vi "IR Opo Main.vi"() -> ()   [LabVIEW 2016] (continued)
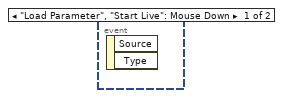
[diagram p2: hidden frame]
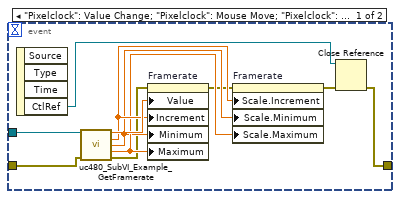
[diagram p3: hidden frame]
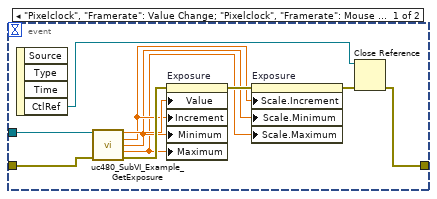
[diagram p4: hidden frame]
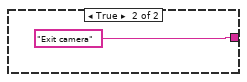
[diagram p5: hidden frame]
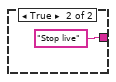
[diagram p6: hidden frame]
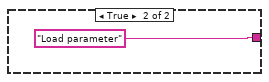
[diagram p7: hidden frame]
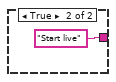
[diagram p8: hidden frame]
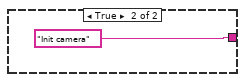
[diagram p9: hidden frame]
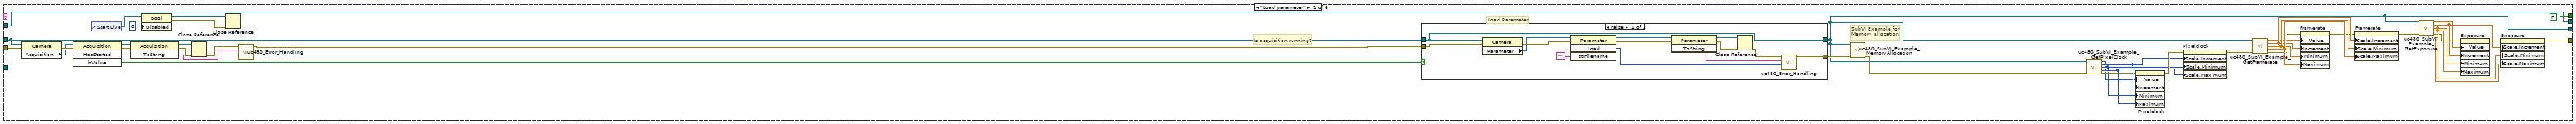
[diagram p10: hidden frame]
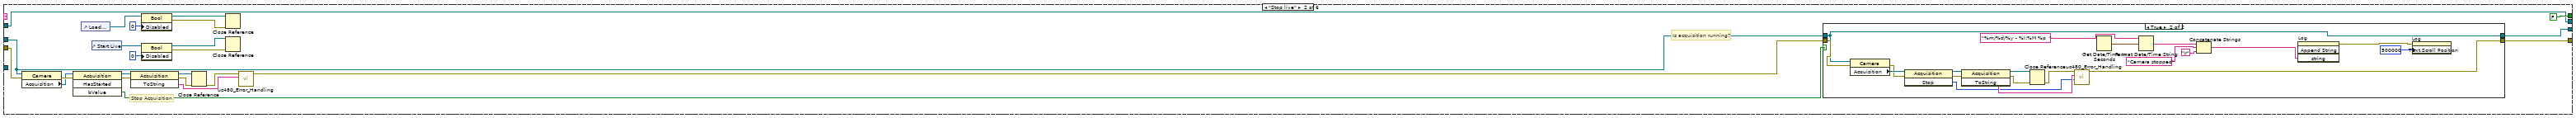
[diagram p12: hidden frame]
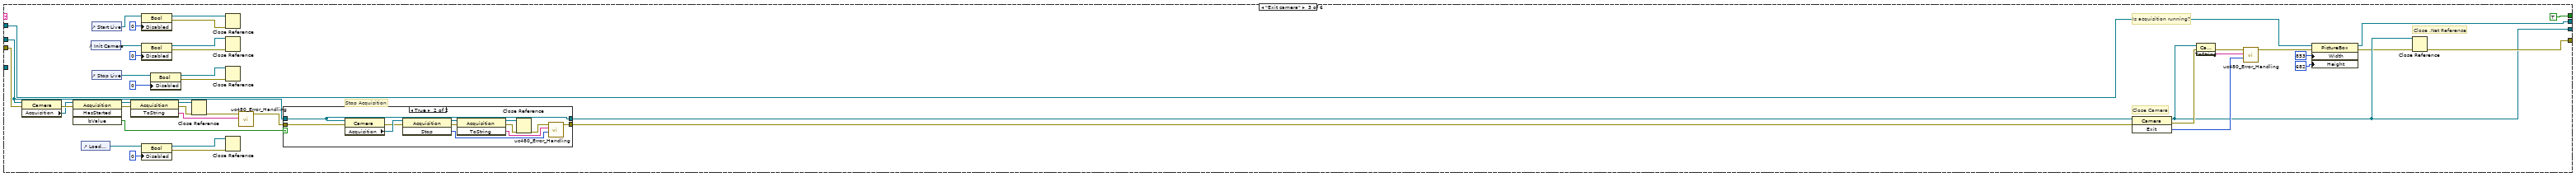
[diagram p14: hidden frame]
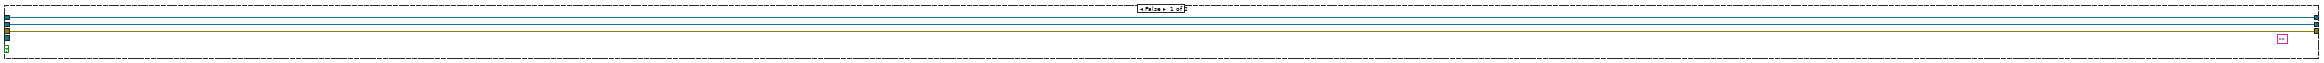
[diagram p16: hidden frame]
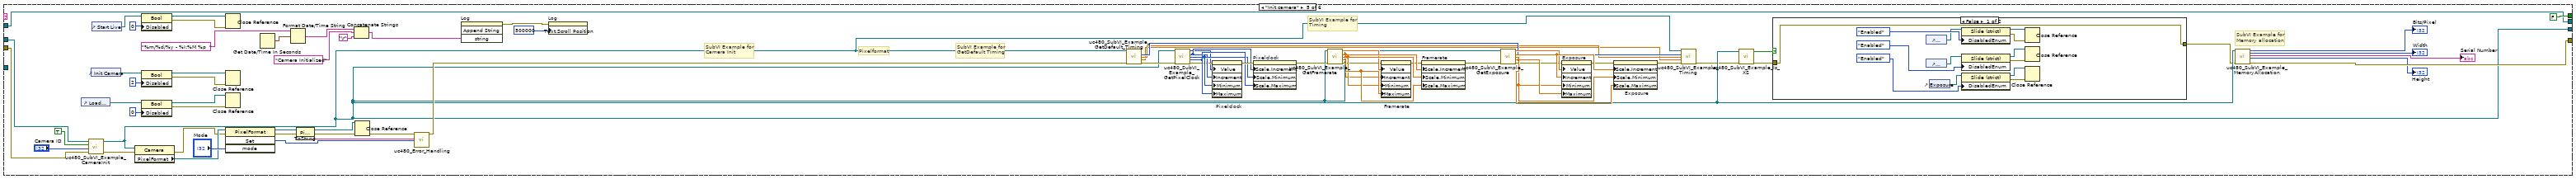
[diagram p18: hidden frame]
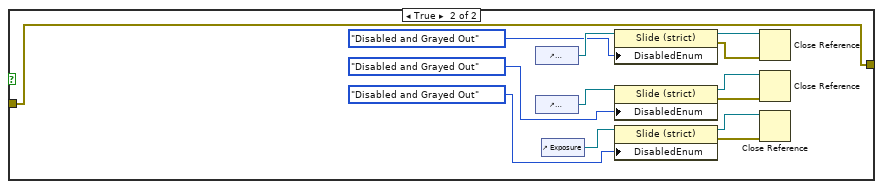
[diagram p19: hidden frame]
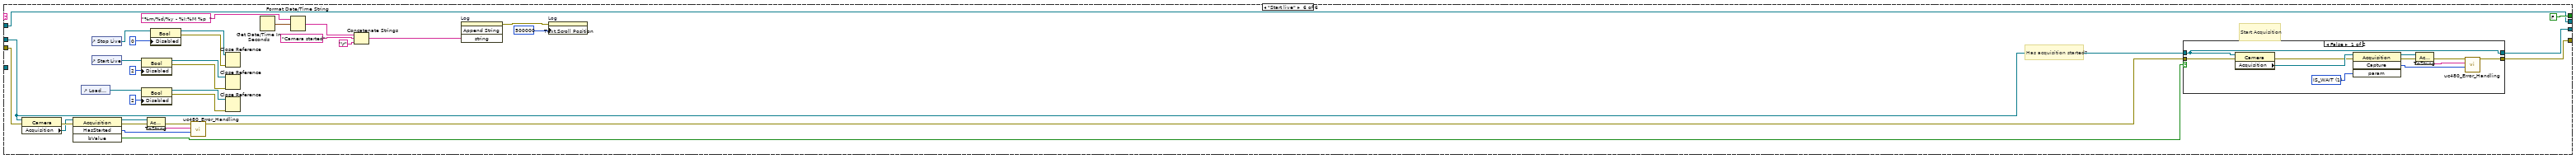
[diagram p20: hidden frame]
            n585 = call <vilib>:"Check if File or Folder Exists.vi"("path"=w1404) -> ("file or folder exists?"=w1403:bool, "dup path"=w1402:path)  [unwired: 8 in, 1 out]
            n586 = case shown="True" w1403 {
              tunnel: w1402 -> [w1414 w1415]
              tunnel: [w1413 w1415] -> w1401
              frame False {
                n587 = Create Folder(path (use dialog)=w1414) -> (created path=w1413:path)  [unwired: 2 in, 2 out]
              }
              frame True {
              }
            }
            n588 = Get Date/Time In Seconds() -> (seconds since 1Jan1904=w1398:timestamp)
            n589 = Format Date/Time String(time format string (%c)="%d%m%y %I-%M %p ", seconds (now)=w1398) -> (date/time string=w1397:string)  [unwired: 1 in]
            n590 = Concatenate Strings(w1397, " - saved ROI.tiff" ("string")) -> (w1395:string)
            n591 = Build Path(base path=w1401, name or relative path=w1395) -> (appended path=w1400:path)
            n592 = call-poly "IMAQ Write File 2"("File Path"=w1400, "Image"=w1408) -> ()  [unwired: 8 in, 2 out]
          }
        }
      }
      event "Load ROI": Value Change {
        n593 = event-data() -> ()  [unwired: 1 in, 6 out]
        n594 = case shown="True" "Load ROI" {
          frame False {
          }
          frame True {
            n595 = call "File Dialog"("prompt"="Select an ROI file..." ("pattern label"), "pattern (all files)"="*.jpg;*.bmp;*.jpeg;*.tif;*.tiff;*.png", "pattern label"="ROI files") -> ("selected path"=w1417:path, "cancelled"=w1418:bool)  [unwired: 9 in, 2 out]
            n596 = case shown="False" w1418 {
              tunnel: w1417 -> [w1429 _]
              frame False {
                n597 = call "IMAQ Create"("Image Name"="untitled") -> ("New Image"=w1431:T2)  [unwired: 4 in, 1 out]
                n598 = call "IMAQ ReadFile"("File Path"=w1429, "Image"=w1431) -> ("Image Out"=w1430:T2)  [unwired: 5 in, 4 out]
                n599 = call "IMAQ MaskToROI"("Image"=w1430) -> ("ROI Descriptor"=w1422:T13)  [unwired: 6 in, 2 out]
                n600 = Unbundle By Name(w1422) -> ("Contours"=w1427:T14)  [unwired: 1 out]
                n601 = Index Array(array=w1427) -> (element=w1428:T15)  [unwired: 1 in]
                n602 = Bundle By Name(cluster=w1428, "Type"=u32 6) -> (w1426:T15)
                n603 = Replace Array Subset(array=w1427, new element=w1426) -> (w1425:T14)  [unwired: 1 in]
                n604 = Bundle By Name(cluster=w1422, "Contours"=w1425) -> (w1423:T13)
                n605 = property on="Source" class="ImageControl"("ROI"=w1423) -> ()  [unwired: 2 in, 2 out]
              }
              frame True {
              }
            }
          }
        }
      }
      event "Axes Manual Control": Value Change {
        n606 = event-data() -> ()  [unwired: 1 in, 6 out]
        n607 = case shown="True" "Axes Manual Control" {
          tunnel: w1435 -> [_ w1447]
          tunnel: w1434 -> [_ w1446]
          tunnel: w1433 -> [_ w1445]
          frame False {
          }
          frame True {
            n608 = flat-sequence {
              tunnel: w1447 -> [w1457]
              tunnel: w1446 -> [w1456]
              tunnel: w1445 -> [w1455]
              tunnel: [w1457] -> w1444
              tunnel: [w1456] -> w1443
              tunnel: [w1455] -> w1442
              tunnel: [w1454] -> w1441
              tunnel: [w1453] -> w1440
              tunnel: [w1452] -> w1439
              tunnel: [w1451] -> w1438
              tunnel: w1444 -> [w1500]
              tunnel: w1443 -> [w1499]
              tunnel: w1442 -> [w1498]
              tunnel: w1441 -> [w1493]
              tunnel: w1440 -> [w1492]
              tunnel: w1439 -> [w1483]
              tunnel: w1438 -> [w1482]
              frame #0 {
                n609 = call <userlib>:"Open TCP-IP.vi"("IP address"=w1457) -> ("error out"=w1449:errorcluster, "Connection ID"=w1458:T9)  [unwired: 8 in, 1 out]
                n610 = call <vilib>:"Simple Error Handler.vi"("error in (no error)"=w1449) -> ("error?"=w1448:bool, "error out"=w1450:errorcluster)  [unwired: 4 in, 3 out]
                n611 = case shown="True" w1448 {
                  tunnel: w1458 -> [w1473 _]
                  tunnel: w1450 -> [w1472 _]
                  tunnel: w1456 -> [w1469 _]
                  tunnel: w1455 -> [w1468 _]
                  tunnel: [w1467 w1477] -> w1454
                  tunnel: [w1466 w1477] -> w1453
                  tunnel: [w1462 w1476] -> w1452
                  tunnel: [w1461 w1476] -> w1451
                  frame False {
                    n612 = call "Get Stages Status.vi"("error in (no error)"=w1472, "Group Name (250 c max)"=w1469, "connection ID in"=w1473) -> ("error out"=w1471:errorcluster, "XPS error out"=w1470:errorcluster, "Group Status String"=w1466:string, "connection ID out"=w1465:T9, "Status"=w1461:i32)  [unwired: 4 in]
                    n613 = call "Get Stages Status.vi"("error in (no error)"=w1471, "XPS error in (no error)"=w1470, "Group Name (250 c max)"=w1468, "connection ID in"=w1465) -> ("error out"=w1475:errorcluster, "XPS error out"=w1464:errorcluster, "Group Status String"=w1467:string, "connection ID out"=w1474:T9, "Status"=w1462:i32)  [unwired: 3 in]
                    n614 = call <vilib>:"Simple Error Handler.vi"("error source (\" \")"="Axis manual control check" ("error source (\" \")"), "error in (no error)"=w1464) -> ()  [unwired: 3 in, 5 out]
                    n615 = call <userlib>:"Close TCP-IP.vi"("error in (no error)"=w1475, "connection ID in"=w1474) -> ("Error out"=w1463:errorcluster)  [unwired: 9 in]
                    n616 = call <vilib>:"Simple Error Handler.vi"("error source (\" \")"="TCP close Axis manual control check" ("error source (\" \")"), "error in (no error)"=w1463) -> ()  [unwired: 3 in, 5 out]
                  }
                  frame True {
                    w1476 = 0
                    w1477 = ""
                  }
                }
              }
              frame #1 {
                w1486 = 47 ("y")
                w1487 = "Ready"
                n617 = String Subset(string=w1492, offset (0)=0, length (rest)=5 ("length (rest)")) -> (substring=w1489:string)
                n618 = String Subset(string=w1493, offset (0)=0, length (rest)=5 ("length (rest)")) -> (substring=w1488:string)
                n619 = Equal?(x=w1489, y=w1487) -> (x = y?=w1490:bool)
                n620 = Equal?(x=w1487, y=w1488) -> (x = y?=w1491:bool)
                n621 = Equal?(x=w1486, y=w1482) -> (x = y?=w1484:bool)
                n622 = Equal?(x=w1483, y=w1486) -> (x = y?=w1485:bool)
                n623 = And(x=w1485, y=w1484) -> (x .and. y?=w1479:bool)
                n624 = And(x=w1490, y=w1491) -> (x .and. y?=w1480:bool)
                n625 = Not(x=w1479) -> (.not. x?=w1478:bool)
                n626 = And(x=w1480, y=w1478) -> (x .and. y?=w1481:bool)
                n627 = case shown="True" w1481 {
                  tunnel: w1500 -> [_ w1506]
                  tunnel: w1499 -> [_ w1505]
                  tunnel: w1498 -> [_ w1504]
                  tunnel: w1478 -> [w1501 _]
                  frame False {
                    n628 = case shown="False" w1501 {
                      frame False {
                        n629 = One Button Dialog(message="One or more axis already in jogging position") -> ()  [unwired: 1 in, 1 out]
                      }
                      frame True {
                        n630 = One Button Dialog(message="Axes are not ready") -> ()  [unwired: 1 in, 1 out]
                      }
                    }
                  }
                  frame True {
                    n631 = call "XPS_LTA_HS_Jogger.vi"("Axis 2"=w1504, "Axis 1"=w1505, "Controller Address"=w1506) -> ()  [unwired: 8 in]
                  }
                }
              }
            }
          }
        }
      }
      event "Home Axes": Value Change {
        n632 = event-data() -> ()  [unwired: 1 in, 6 out]
        n633 = flat-sequence {
          tunnel: w1513 -> [w1519]
          tunnel: w1514 -> [w1520]
          tunnel: w1515 -> [w1521]
          tunnel: "Home Axes" -> [w1522]
          tunnel: [w1522] -> w1511
          tunnel: [w1521] -> w1510
          tunnel: [w1520] -> w1509
          tunnel: [w1519] -> w1508
          tunnel: [w1518] -> w1507
          tunnel: [w1526] -> w1512
          tunnel: w1511 -> [w1524]
          tunnel: w1510 -> [w1529]
          tunnel: w1509 -> [w1527]
          tunnel: w1508 -> [w1528]
          tunnel: w1507 -> [w1525]
          tunnel: [w1608] -> w1516
          tunnel: w1512 -> [w1607]
          frame #0 {
            n634 = call "Display Message to User"() -> ("OK"=w1518:bool)  [unwired: 10 in, 1 out]
          }
          frame #1 {
            n635 = And(x=w1524, y=w1525) -> (x .and. y?=w1523:bool)
            n636 = case shown="True" w1523 {
              tunnel: w1529 -> [_ w1545]
              tunnel: w1527 -> [_ w1546]
              tunnel: w1528 -> [_ w1543]
              tunnel: w1527 -> [_ w1544]
              tunnel: [FALSE w1536] -> w1526
              frame False {
              }
              frame True {
                w1542 = 47 ("y")
                w1558 = "Ready"
                n637 = call <userlib>:"Open TCP-IP.vi"("IP address"=w1545) -> ("error out"=w1531:errorcluster, "Connection ID"=w1549:T9)  [unwired: 8 in, 1 out]
                n638 = call <vilib>:"Simple Error Handler.vi"("error in (no error)"=w1531) -> ("error?"=w1533:bool, "error out"=w1532:errorcluster)  [unwired: 4 in, 3 out]
                n639 = case shown="False" w1533 {
                  tunnel: w1532 -> [w1572 _]
                  tunnel: w1549 -> [w1571 _]
                  tunnel: [w1568 w1577] -> w1548
                  tunnel: [w1567 w1577] -> w1547
                  tunnel: w1546 -> [w1566 _]
                  tunnel: w1543 -> [w1565 _]
                  tunnel: [w1562 w1576] -> w1541
                  tunnel: [w1561 w1576] -> w1540
                  frame False {
                    n640 = call "Get Stages Status.vi"("error in (no error)"=w1572, "Group Name (250 c max)"=w1566, "connection ID in"=w1571) -> ("error out"=w1573:errorcluster, "XPS error out"=w1574:errorcluster, "Group Status String"=w1568:string, "connection ID out"=w1575:T9, "Status"=w1561:i32)  [unwired: 4 in]
                    n641 = call "Get Stages Status.vi"("error in (no error)"=w1573, "XPS error in (no error)"=w1574, "Group Name (250 c max)"=w1565, "connection ID in"=w1575) -> ("error out"=w1569:errorcluster, "XPS error out"=w1564:errorcluster, "Group Status String"=w1567:string, "connection ID out"=w1570:T9, "Status"=w1562:i32)  [unwired: 3 in]
                    n642 = call <vilib>:"Simple Error Handler.vi"("error source (\" \")"="home axis check" ("error source (\" \")"), "error in (no error)"=w1564) -> ()  [unwired: 3 in, 5 out]
                    n643 = call <userlib>:"Close TCP-IP.vi"("error in (no error)"=w1569, "connection ID in"=w1570) -> ("Error out"=w1563:errorcluster)  [unwired: 9 in]
                    n644 = call <vilib>:"Simple Error Handler.vi"("error source (\" \")"="TCP close home axis check" ("error source (\" \")"), "error in (no error)"=w1563) -> ()  [unwired: 3 in, 5 out]
                  }
                  frame True {
                    w1576 = 0
                    w1577 = ""
                  }
                }
                n645 = Equal?(x=w1542, y=w1540) -> (x = y?=w1539:bool)
                n646 = Equal?(x=w1541, y=w1542) -> (x = y?=w1538:bool)
                n647 = String Subset(string=w1548, offset (0)=0, length (rest)=5 ("length (rest)")) -> (substring=w1556:string)
                n648 = String Subset(string=w1547, offset (0)=0, length (rest)=5 ("length (rest)")) -> (substring=w1557:string)
                n649 = Equal?(x=w1556, y=w1558) -> (x = y?=w1555:bool)
                n650 = Equal?(x=w1558, y=w1557) -> (x = y?=w1554:bool)
                n651 = And(x=w1538, y=w1539) -> (x .and. y?=w1534:bool)
                n652 = Not(x=w1534) -> (.not. x?=w1535:bool)
                n653 = And(x=w1555, y=w1554) -> (x .and. y?=w1537:bool)
                n654 = And(x=w1537, y=w1535) -> (x .and. y?=w1536:bool)
                n655 = case shown="True" w1536 {
                  tunnel: w1545 -> [_ w1587]
                  tunnel: w1544 -> [_ w1586]
                  tunnel: w1543 -> [_ w1585]
                  tunnel: w1534 -> [w1578 _]
                  frame False {
                    n656 = case shown="True" w1578 {
                      frame False {
                        n657 = One Button Dialog(message="Axes are not ready") -> ()  [unwired: 1 in, 1 out]
                      }
                      frame True {
                        n658 = One Button Dialog(message="One or more axis are in jogging mode") -> ()  [unwired: 1 in, 1 out]
                      }
                    }
                  }
                  frame True {
                    n659 = call <userlib>:"Open TCP-IP.vi"("IP address"=w1587) -> ("error out"=w1603:errorcluster, "Connection ID"=w1604:T9)  [unwired: 8 in, 1 out]
                    n660 = call <userlib>:"Group Kill.vi"("error in (no error)"=w1603, "Group Name (250 c max)"=w1586, "connection ID in"=w1604) -> ("error out"=w1601:errorcluster, "XPS error out"=w1602:errorcluster, "connection ID out"=w1598:T9)  [unwired: 6 in]
                    n661 = call <userlib>:"Group Initialize.vi"("error in (no error)"=w1601, "XPS error in (no error)"=w1602, "Group Name (250 c max)"=w1586, "connection ID in"=w1598) -> ("error out"=w1599:errorcluster, "XPS error out"=w1600:errorcluster, "connection ID out"=w1597:T9)  [unwired: 5 in]
                    n662 = call <userlib>:"Group Home Search.vi"("error in (no error)"=w1599, "XPS error in (no error)"=w1600, "Group Name (250 c max)"=w1586, "connection ID in"=w1597) -> ("error out"=w1588:errorcluster, "XPS error out"=w1589:errorcluster, "connection ID out"=w1596:T9)  [unwired: 5 in]
                    n663 = call <userlib>:"Group Kill.vi"("error in (no error)"=w1588, "XPS error in (no error)"=w1589, "Group Name (250 c max)"=w1585, "connection ID in"=w1596) -> ("error out"=w1590:errorcluster, "XPS error out"=w1591:errorcluster, "connection ID out"=w1595:T9)  [unwired: 5 in]
                    n664 = call <userlib>:"Group Initialize.vi"("error in (no error)"=w1590, "XPS error in (no error)"=w1591, "Group Name (250 c max)"=w1585, "connection ID in"=w1595) -> ("error out"=w1592:errorcluster, "XPS error out"=w1593:errorcluster, "connection ID out"=w1594:T9)  [unwired: 5 in]
                    n665 = call <userlib>:"Group Home Search.vi"("error in (no error)"=w1592, "XPS error in (no error)"=w1593, "Group Name (250 c max)"=w1585, "connection ID in"=w1594) -> ("error out"=w1605:errorcluster, "XPS error out"=w1584:errorcluster, "connection ID out"=w1606:T9)  [unwired: 5 in]
                    n666 = call <vilib>:"Simple Error Handler.vi"("error source (\" \")"="home axis " ("error source (\" \")"), "error in (no error)"=w1584) -> ()  [unwired: 3 in, 5 out]
                    n667 = call <userlib>:"Close TCP-IP.vi"("error in (no error)"=w1605, "connection ID in"=w1606) -> ("Error out"=w1583:errorcluster)  [unwired: 9 in]
                    n668 = call <vilib>:"Simple Error Handler.vi"("error source (\" \")"="TCP close home axis " ("error source (\" \")"), "error in (no error)"=w1583) -> ()  [unwired: 3 in, 5 out]
                  }
                }
              }
            }
          }
          frame #2 {
            n669 = case shown="True" w1607 {
              tunnel: ["" ("StringOut") "Axes have been moved to home position" ("StringOut")] -> w1608
              frame False {
              }
              frame True {
              }
            }
          }
        }
      }
      event "Transparency": Value Change {
        n670 = event-data() -> ()  [unwired: 1 in, 6 out]
        n671 = control-ref of="This VI"() -> (w1612:refnum<vi>)
        n672 = property class="VI"(reference=w1612, "FP:Transparency"="Transparency") -> ()  [unwired: 1 in, 2 out]
      }
      event "Capture": Value Change {
        w1613 = 47 ("y")
        w1639 = "Ready"
        n673 = event-data() -> ()  [unwired: 1 in, 6 out]
        n674 = call <userlib>:"Open TCP-IP.vi"("IP address"=w1627) -> ("error out"=w1616:errorcluster, "Connection ID"=w1630:T9)  [unwired: 8 in, 1 out]
        n675 = call <vilib>:"Simple Error Handler.vi"("error in (no error)"=w1616) -> ("error?"=w1614:bool, "error out"=w1615:errorcluster)  [unwired: 4 in, 3 out]
        n676 = case shown="False" w1614 {
          tunnel: w1615 -> [w1653 _]
          tunnel: w1630 -> [w1652 _]
          tunnel: [w1649 w1657] -> w1629
          tunnel: [w1648 w1657] -> w1628
          tunnel: w1626 -> [w1647 _]
          tunnel: w1625 -> [w1646 _]
          tunnel: [w1644 w1658] -> w1624
          tunnel: [w1643 w1658] -> w1623
          frame False {
            n677 = call "Get Stages Status.vi"("error in (no error)"=w1653, "Group Name (250 c max)"=w1647, "connection ID in"=w1652) -> ("error out"=w1654:errorcluster, "XPS error out"=w1655:errorcluster, "Group Status String"=w1649:string, "connection ID out"=w1656:T9, "Status"=w1643:i32)  [unwired: 4 in]
            n678 = call "Get Stages Status.vi"("error in (no error)"=w1654, "XPS error in (no error)"=w1655, "Group Name (250 c max)"=w1646, "connection ID in"=w1656) -> ("error out"=w1650:errorcluster, "XPS error out"=w1645:errorcluster, "Group Status String"=w1648:string, "connection ID out"=w1651:T9, "Status"=w1644:i32)  [unwired: 3 in]
            n679 = call <vilib>:"Simple Error Handler.vi"("error source (\" \")"="Capture check" ("error source (\" \")"), "error in (no error)"=w1645) -> ()  [unwired: 3 in, 5 out]
            n680 = call <userlib>:"Close TCP-IP.vi"("error in (no error)"=w1650, "connection ID in"=w1651) -> ("Error out"=w1641:errorcluster)  [unwired: 9 in]
            n681 = call <vilib>:"Simple Error Handler.vi"("error in (no error)"=w1641) -> ()  [unwired: 4 in, 5 out]
          }
          frame True {
            w1658 = 0
            w1657 = ""
          }
        }
        n682 = Equal?(x=w1624, y=w1613) -> (x = y?=w1622:bool)
        n683 = Equal?(x=w1613, y=w1623) -> (x = y?=w1621:bool)
        n684 = String Subset(string=w1629, offset (0)=0, length (rest)=5 ("length (rest)")) -> (substring=w1637:string)
        n685 = String Subset(string=w1628, offset (0)=0, length (rest)=5 ("length (rest)")) -> (substring=w1638:string)
        n686 = Equal?(x=w1637, y=w1639) -> (x = y?=w1636:bool)
        n687 = Equal?(x=w1639, y=w1638) -> (x = y?=w1635:bool)
        n688 = And(x=w1622, y=w1621) -> (x .and. y?=w1618:bool)
        n689 = Not(x=w1618) -> (.not. x?=w1617:bool)
        n690 = And(x=w1636, y=w1635) -> (x .and. y?=w1620:bool)
        n691 = And(x=w1620, y=w1617) -> (x .and. y?=w1619:bool)
        n692 = case shown="True" w1619 {
          tunnel: ["" w1666] -> w1640
          tunnel: w1627 -> [_ w1665]
          tunnel: w1625 -> [_ w1664]
          tunnel: w1626 -> [_ w1663]
          tunnel: w1618 -> [w1659 _]
          frame False {
            n693 = case shown="True" w1659 {
              frame False {
                n694 = One Button Dialog(message="Axes are not ready") -> ()  [unwired: 1 in, 1 out]
              }
              frame True {
                n695 = One Button Dialog(message="One or more axis are in jogging mode") -> ()  [unwired: 1 in, 1 out]
              }
            }
          }
          frame True {
            n696 = flat-sequence {
              tunnel: [w1687] -> w1678
              tunnel: [w1686] -> w1677
              tunnel: [w1685] -> w1676
              tunnel: [w1684] -> w1675
              tunnel: [w1683] -> w1674
              tunnel: [w1682] -> w1673
              tunnel: [w1681] -> w1672
              tunnel: w1665 -> [w1681]
              tunnel: w1664 -> [w1680]
              tunnel: w1663 -> [w1679]
              tunnel: w1678 -> [w1707]
              tunnel: w1677 -> [w1698]
              tunnel: w1676 -> [w1699]
              tunnel: w1675 -> [w1705]
              tunnel: w1674 -> [w1704]
              tunnel: [w1697] -> w1671
              tunnel: w1673 -> [w1697]
              tunnel: [w1696] -> w1670
              tunnel: w1672 -> [w1696]
              tunnel: [w1709] -> w1669
              tunnel: w1671 -> [w1709]
              tunnel: [w1708] -> w1668
              tunnel: w1670 -> [w1708]
              tunnel: w1669 -> [w1717]
              tunnel: w1668 -> [w1722]
              tunnel: [w1716] -> w1667
              tunnel: [w1731] -> w1666
              tunnel: w1667 -> [w1728]
              frame #0 {
                w1692 = ".Pos"
                n697 = local read "Axis Initial Parameters"() -> (w1682:T1)
                n698 = Concatenate Strings(w1679, w1692) -> (w1686:string)
                n699 = call <userlib>:"Open TCP-IP.vi"("IP address"=w1681) -> ("error out"=w1688:errorcluster, "Connection ID"=w1693:T9)  [unwired: 5 in, 4 out]
                n700 = Concatenate Strings(w1680, w1692) -> (w1685:string)
                n701 = call <userlib>:"Positioner SGamma Parameters Set.vi"("SGamma Parameters"=w1682, "error in (no error)"=w1688, "Positioner Name (250 c max)"=w1686, "connection ID in"=w1693) -> ("error out"=w1689:errorcluster, "XPS error out"=w1690:errorcluster, "connection ID out"=w1691:T9)  [unwired: 5 in]
                n702 = call <userlib>:"Positioner SGamma Parameters Set.vi"("SGamma Parameters"=w1682, "error in (no error)"=w1689, "XPS error in (no error)"=w1690, "Positioner Name (250 c max)"=w1685, "connection ID in"=w1691) -> ("error out"=w1684:errorcluster, "XPS error out"=w1683:errorcluster, "connection ID out"=w1687:T9)  [unwired: 4 in]
              }
              frame #1 {
                n703 = local read "Axis 2 Offset"() -> (w1695:dbl)
                n704 = local read "Axis 1 Offset"() -> (w1694:dbl)
                n705 = call <userlib>:"Single Axis Group Move Relative.vi"("Target Displacement (units)"=w1695, "error in (no error)"=w1705, "XPS error in (no error)"=w1704, "SingleAxis Group  Name (250 c max)"=w1698, "connection ID in"=w1707) -> ("error out"=w1702:errorcluster, "XPS error out"=w1703:errorcluster, "connection ID out"=w1706:T9)  [unwired: 4 in]
                n706 = call <userlib>:"Single Axis Group Move Relative.vi"("Target Displacement (units)"=w1694, "error in (no error)"=w1702, "XPS error in (no error)"=w1703, "SingleAxis Group  Name (250 c max)"=w1699, "connection ID in"=w1706) -> ("error out"=w1700:errorcluster, "connection ID out"=w1701:T9)  [unwired: 4 in, 1 out]
                n707 = call <userlib>:"Close TCP-IP.vi"("error in (no error)"=w1700, "connection ID in"=w1701) -> ()  [unwired: 9 in, 1 out]
              }
              frame #2 {
                n708 = Wait (ms)(milliseconds to wait=u32 1000) -> ()  [unwired: 1 out]
              }
              frame #3 {
                n709 = local read "Speed (µm/s)"() -> (w1721:i32)
                n710 = local read "Processi time (sec)"() -> (w1715:i32)
                n711 = local read "Laser on/off array"() -> (w1725:bool[][])
                n712 = local read "Commands array"() -> (w1726:string[][])
                n713 = local read "ROI Area \n(mm2)"() -> (w1713:dbl)
                n714 = local read "Laser Com Delay"() -> (w1712:i32)
                n715 = local read "VISA Laser port"() -> (w1711:string)
                n716 = Divide(x=w1721, y=1000) -> (x/y=w1718:dbl)
                n717 = call "IR_OPO_Capture_V2.vi"("Commands array"=w1726, "XPS_Address"=w1722, "VISA resource name"=w1711, "laser array index"=0, "Process time"=w1715, "Axis Speed"=w1718, "Laser on/off array"=w1725, "stop"=FALSE ("STOP CAPTURE"), "delay before read (ms)"=w1712, "Axis Initial Parameters"=w1717, "ROI Area \n(mm2)"=w1713, "OPO on?"=TRUE, "Acceleration (units/seconds²)"="Acceleration \n(mm/s²)") -> ("Elapsed time"=w1716:dbl)  [unwired: 6 in]
              }
              frame #4 {
                n718 = Number To Decimal String(number=w1728) -> (decimal integer string=w1727:string)  [unwired: 1 in]
                n719 = Concatenate Strings("Capture completed in " ("StringOut"), w1727, " seconds" ("string")) -> (w1731:string)
              }
            }
          }
        }
      }
      event "Microscope/Capture \nstatus button": Value Change {
        w1751 = 47 ("y")
        w1764 = "Ready"
        n720 = event-data() -> ()  [unwired: 1 in, 6 out]
        n721 = call <userlib>:"Open TCP-IP.vi"("IP address"=w1732) -> ("error out"=w1767:errorcluster, "Connection ID"=w1768:T9)  [unwired: 8 in, 1 out]
        n722 = call <vilib>:"Simple Error Handler.vi"("error in (no error)"=w1767) -> ("error?"=w1765:bool, "error out"=w1766:errorcluster)  [unwired: 4 in, 3 out]
        n723 = case shown="False" w1765 {
          tunnel: w1768 -> [w1844 _]
          tunnel: [w1841 w1848] -> w1750
          tunnel: [w1840 w1848] -> w1749
          tunnel: w1744 -> [w1839 _]
          tunnel: w1745 -> [w1838 _]
          tunnel: [w1836 w1849] -> w1748
          tunnel: [w1835 w1849] -> w1747
          tunnel: w1766 -> [w1832 _]
          frame False {
            n724 = call "Get Stages Status.vi"("error in (no error)"=w1832, "Group Name (250 c max)"=w1839, "connection ID in"=w1844) -> ("error out"=w1845:errorcluster, "XPS error out"=w1846:errorcluster, "Group Status String"=w1841:string, "connection ID out"=w1847:T9, "Status"=w1835:i32)  [unwired: 4 in]
            n725 = call "Get Stages Status.vi"("error in (no error)"=w1845, "XPS error in (no error)"=w1846, "Group Name (250 c max)"=w1838, "connection ID in"=w1847) -> ("error out"=w1842:errorcluster, "XPS error out"=w1837:errorcluster, "Group Status String"=w1840:string, "connection ID out"=w1843:T9, "Status"=w1836:i32)  [unwired: 3 in]
            n726 = call <vilib>:"Simple Error Handler.vi"("error source (\" \")"="Axes check" ("error source (\" \")"), "error in (no error)"=w1837) -> ()  [unwired: 3 in, 5 out]
            n727 = call <userlib>:"Close TCP-IP.vi"("error in (no error)"=w1842, "connection ID in"=w1843) -> ("Error out"=w1833:errorcluster)  [unwired: 9 in]
            n728 = call <vilib>:"Simple Error Handler.vi"("error in (no error)"=w1833) -> ()  [unwired: 4 in, 5 out]
          }
          frame True {
            w1849 = 0
            w1848 = ""
          }
        }
        n729 = Equal?(x=w1748, y=w1751) -> (x = y?=w1755:bool)
        n730 = Equal?(x=w1751, y=w1747) -> (x = y?=w1754:bool)
        n731 = String Subset(string=w1750, offset (0)=0, length (rest)=5 ("length (rest)")) -> (substring=w1762:string)
        n732 = String Subset(string=w1749, offset (0)=0, length (rest)=5 ("length (rest)")) -> (substring=w1763:string)
        n733 = case shown="False" "Microscope/Capture \nstatus button" {
          tunnel: ["capture " "microscope "] -> w1737
          frame False {
          }
          frame True {
          }
        }
        n734 = Equal?(x=w1762, y=w1764) -> (x = y?=w1761:bool)
        n735 = Equal?(x=w1764, y=w1763) -> (x = y?=w1760:bool)
        n736 = And(x=w1755, y=w1754) -> (x .and. y?=w1746:bool)
        n737 = Not(x=w1746) -> (.not. x?=w1752:bool)
        n738 = And(x=w1761, y=w1760) -> (x .and. y?=w1753:bool)
        n739 = And(x=w1753, y=w1752) -> (x .and. y?=w1735:bool)
        n740 = Concatenate Strings("Do you want to move the axis to the " ("message"), w1737, "position?" ("string")) -> (w1736:string)
        n741 = Two Button Dialog(message=w1736, 1:"No" ("F button name (\"Cancel\")"), 2:"Yes" ("T button name (\"OK\")")) -> (T button?=w1734:bool)
        n742 = And(x=w1735, y=w1734) -> (x .and. y?=w1733:bool)
        n743 = case shown="True" w1733 {
          tunnel: "Microscope/Capture \nstatus button" -> [_ w1777]
          tunnel: w1746 -> [w1772 _]
          tunnel: w1745 -> [_ w1785]
          tunnel: w1744 -> [_ w1784]
          tunnel: [_ w1783] -> w1743
          tunnel: w1734 -> [w1771 _]
          tunnel: w1732 -> [_ w1776]
          frame False {
            n744 = case shown="True" w1771 {
              tunnel: w1772 -> [_ w1773]
              frame False {
              }
              frame True {
                n745 = case shown="True" w1773 {
                  frame False {
                    n746 = One Button Dialog(message="Axes are not ready") -> ()  [unwired: 1 in, 1 out]
                  }
                  frame True {
                    n747 = One Button Dialog(message="One or more axis are in jogging mode") -> ()  [unwired: 1 in, 1 out]
                  }
                }
              }
            }
          }
          frame True {
            n748 = flat-sequence {
              tunnel: [w1796] -> w1782
              tunnel: [w1795] -> w1781
              tunnel: [w1794] -> w1780
              tunnel: [w1793] -> w1779
              tunnel: [w1792] -> w1778
              tunnel: w1785 -> [w1791]
              tunnel: w1784 -> [w1790]
              tunnel: w1776 -> [w1789]
              tunnel: w1782 -> [w1817]
              tunnel: w1781 -> [w1808]
              tunnel: w1780 -> [w1809]
              tunnel: w1779 -> [w1815]
              tunnel: w1778 -> [w1814]
              tunnel: w1777 -> [w1803]
              tunnel: [w1829] -> w1783
              tunnel: w1777 -> [w1825]
              frame #0 {
                w1801 = ".Pos"
                n749 = local read "Axis Initial Parameters"() -> (w1788:T1)
                n750 = Bundle By Name(cluster=w1788, "Velocity (units/seconds)"=10.0) -> (w1786:T1)
                n751 = call <userlib>:"Open TCP-IP.vi"("IP address"=w1789) -> ("error out"=w1797:errorcluster, "Connection ID"=w1802:T9)  [unwired: 5 in, 4 out]
                n752 = Concatenate Strings(w1790, w1801) -> (w1795:string)
                n753 = call <userlib>:"Positioner SGamma Parameters Set.vi"("SGamma Parameters"=w1788, "error in (no error)"=w1797, "Positioner Name (250 c max)"=w1795, "connection ID in"=w1802) -> ("error out"=w1798:errorcluster, "XPS error out"=w1799:errorcluster, "connection ID out"=w1800:T9)  [unwired: 5 in]
                n754 = Concatenate Strings(w1791, w1801) -> (w1794:string)
                n755 = call <userlib>:"Positioner SGamma Parameters Set.vi"("SGamma Parameters"=w1786, "error in (no error)"=w1798, "XPS error in (no error)"=w1799, "Positioner Name (250 c max)"=w1794, "connection ID in"=w1800) -> ("error out"=w1793:errorcluster, "XPS error out"=w1792:errorcluster, "connection ID out"=w1796:T9)  [unwired: 4 in]
              }
              frame #1 {
                n756 = local read "Y travel"() -> (w1807:dbl)
                n757 = local read "X travel"() -> (w1806:dbl)
                n758 = case shown="False" w1803 {
                  tunnel: w1807 -> [w1819 w1823]
                  tunnel: w1806 -> [w1818 w1822]
                  tunnel: [w1818 w1821] -> w1805
                  tunnel: [w1819 w1820] -> w1804
                  frame False {
                  }
                  frame True {
                    n759 = Negate(x=w1823) -> (-x=w1820:dbl)
                    n760 = Negate(x=w1822) -> (-x=w1821:dbl)
                  }
                }
                n761 = call <userlib>:"Single Axis Group Move Relative.vi"("Target Displacement (units)"=w1805, "error in (no error)"=w1815, "XPS error in (no error)"=w1814, "SingleAxis Group  Name (250 c max)"=w1808, "connection ID in"=w1817) -> ("error out"=w1812:errorcluster, "XPS error out"=w1813:errorcluster, "connection ID out"=w1816:T9)  [unwired: 4 in]
                n762 = call <userlib>:"Single Axis Group Move Relative.vi"("Target Displacement (units)"=w1804, "error in (no error)"=w1812, "XPS error in (no error)"=w1813, "SingleAxis Group  Name (250 c max)"=w1809, "connection ID in"=w1816) -> ("error out"=w1810:errorcluster, "connection ID out"=w1811:T9)  [unwired: 4 in, 1 out]
                n763 = call <userlib>:"Close TCP-IP.vi"("error in (no error)"=w1810, "connection ID in"=w1811) -> ()  [unwired: 9 in, 1 out]
              }
              frame #2 {
                n764 = Wait (ms)(milliseconds to wait=u32 1000) -> ()  [unwired: 1 out]
              }
              frame #3 {
                n765 = case shown="True" w1825 {
                  tunnel: ["capture " ("string") "microscope " ("string")] -> w1826
                  frame False {
                  }
                  frame True {
                  }
                }
                n766 = Concatenate Strings("Stages translated to the " ("StringOut"), w1826, "position." ("string")) -> (w1829:string)
              }
            }
          }
        }
      }
    }
    n767 = Get Date/Time In Seconds() -> (seconds since 1Jan1904=w751:timestamp)
    n768 = Format Date/Time String(time format string (%c)="%m/%d/%y - %I:%M %p  ", seconds (now)=w751) -> (date/time string=w750:string)  [unwired: 1 in]
    n769 = Empty String/Path?(string/path=w747) -> (empty?=w749:bool)
    n770 = Concatenate Strings(w750, w747, "\r") -> (w748:string)
    n771 = case shown="False" w749 {
      tunnel: w748 -> [w757 _]
      frame False {
        n772 = invoke on="Log" class="Str" method="Append String"("string"=w757) -> (error out=w756:errorcluster)  [unwired: 3 in, 3 out]
        n773 = property on="Log" class="Str"(error in=w756, "Text.Scroll Position"=u32 500000) -> ()  [unwired: 1 in, 2 out]
      }
      frame True {
      }
    }
  }
  n774 = control-ref of="Init Camera"() -> (w44:refnum<vi>)
  n775 = control-ref of="Stop Live"() -> (w37:refnum<vi>)
  n776 = property class="Bool"(reference=w37, "Disabled"=u8 2 ("Deaktiviert")) -> (reference out=w28:refnum<vi>, error out=w27:errorcluster)  [unwired: 1 in]
  n777 = property class="Bool"(reference=w44, "Disabled"=u8 0 ("Deaktiviert")) -> (reference out=w32:refnum<vi>, error out=w31:errorcluster)  [unwired: 1 in]
  n778 = Close Reference(reference=w28, error in (no error)=w27) -> ()  [unwired: 1 out]
  n779 = Close Reference(reference=w32, error in (no error)=w31) -> ()  [unwired: 1 out]
  n780 = control-ref of="Load Parameter"() -> (w38:refnum<vi>)
  n781 = control-ref of="Start Live"() -> (w41:refnum<vi>)
  n782 = property class="Bool"(reference=w41, "Disabled"=u8 2 ("Deaktiviert")) -> (reference out=w30:refnum<vi>, error out=w29:errorcluster)  [unwired: 1 in]
  n783 = property class="Bool"(reference=w38, "Disabled"=u8 2 ("Deaktiviert")) -> (reference out=w26:refnum<vi>, error out=w25:errorcluster)  [unwired: 1 in]
  n784 = Close Reference(reference=w30, error in (no error)=w29) -> ()  [unwired: 1 out]
  n785 = Close Reference(reference=w26, error in (no error)=w25) -> ()  [unwired: 1 out]
